vi "cameraTempControllerFrontEnd.vi"(8 "error in (no error)":errorcluster, 11 "CameraTempController":refnum<class "CameraTempController.lvclass">) -> (0 "error out":errorcluster, 3 "CameraTempController out":refnum<class "CameraTempController.lvclass">)   [LabVIEW 2009, in "Hardware.lvlib" / "Channels.lvlib" / "CameraTempController.lvclass"]
uses:
  CameraTempController.lvclass
panel:
  in  "tempControllerBackEndEvents":T1
  in  "tempControllerFrontEndEvents":T2
  out "Ready":bool
  out "Thermometer":dbl(slide)=25.0 scale=-80.0..25.0
  in  "Stop Cooling and Switch off":bool
  out "Status":string
  out "Temperature":dbl
  in  "setPoint":dbl=25.0
  # "On startup, set the desired Camera temperature set point. The Camera will then cool down to that temperature. Once reached the status field will indicate \"TEMP_STABLIZED\".\n\nAt any time you may change the setPoint to any temperature within the range of the Camera. The Camera will then warm up or cool down to that new setPoint, again indicating \"TEMP_STABLIZED\" once reached.\n\nTo Turn off the Camera temperature controller click the \"Stop\" button. This will set the temperature to 10 degrees and warm up the Camera to that temperature. At which point the temperature control program will exit.\n\nNEVER CLICK THE LABVIEW RED BUTTON TO TERMINATE THIS PROGRAM!!!!! This may cause damage to the camera! NEVER CLICK THE WINDOW CLOSE BUTTON too! This app closes itself automatically."
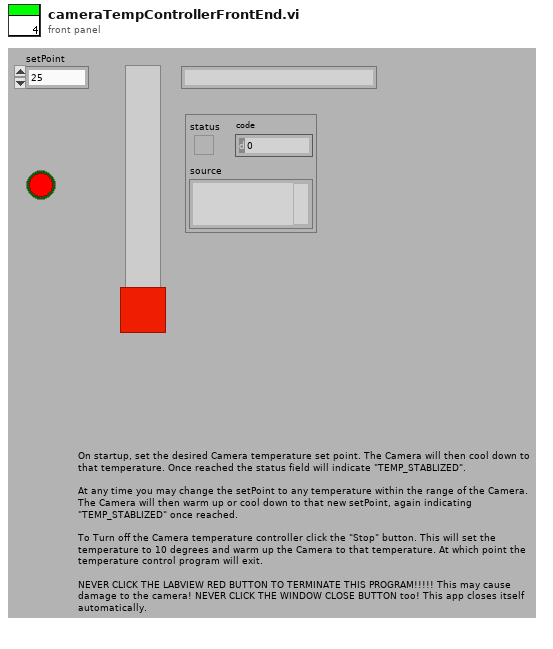
[diagram p1: front panel]
types:
  T1 = cluster{"closeEvent":refnum<user-event>, "temperatureUpdateEvent":refnum<user-event>, "displayErrorEvent":refnum<user-event>, "setPointUpdateEvent":refnum<user-event>}
  T2 = cluster{"newSetPointEvent":refnum<user-event>, "stopCoolingEvent":refnum<user-event>}
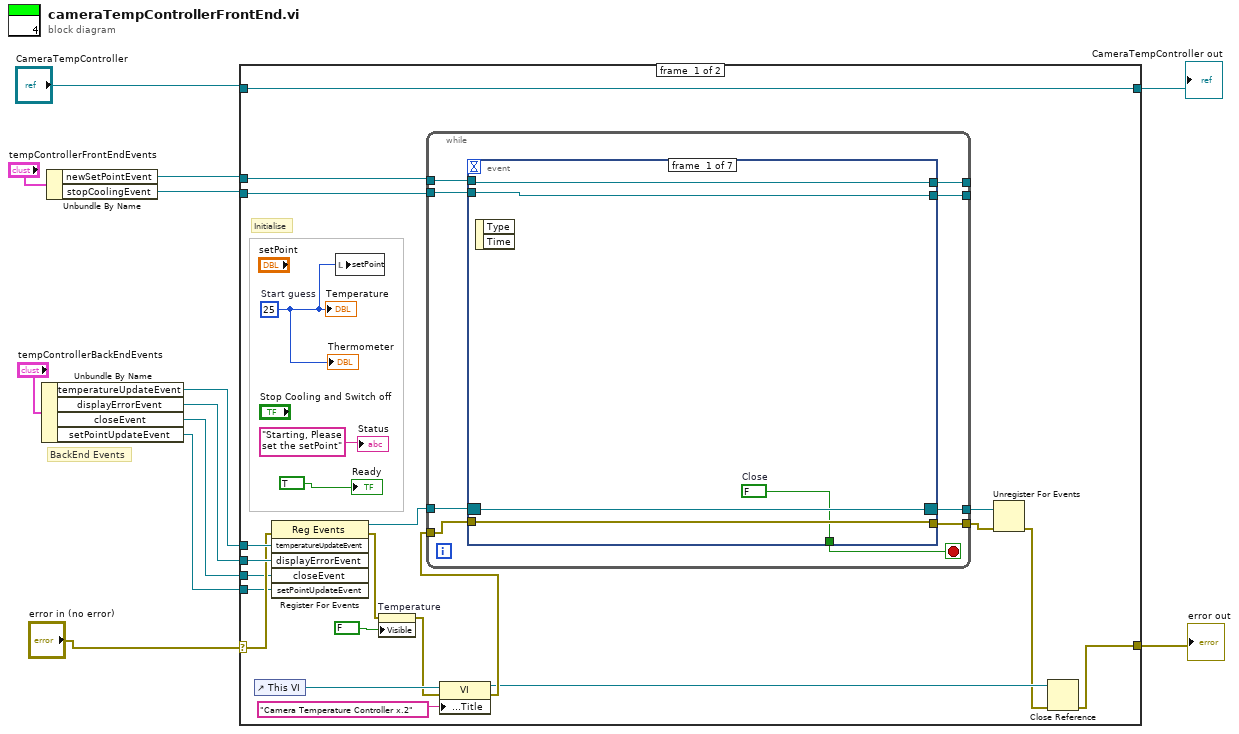
[diagram p0: block diagram]
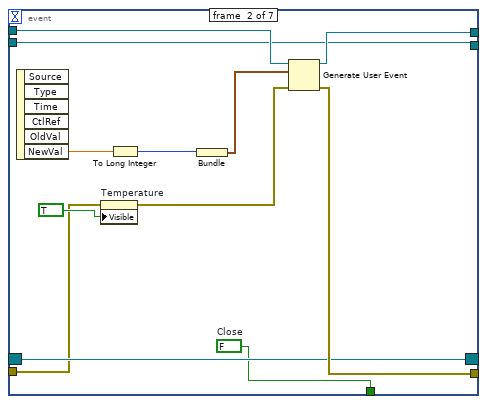
[diagram p2: hidden frame]
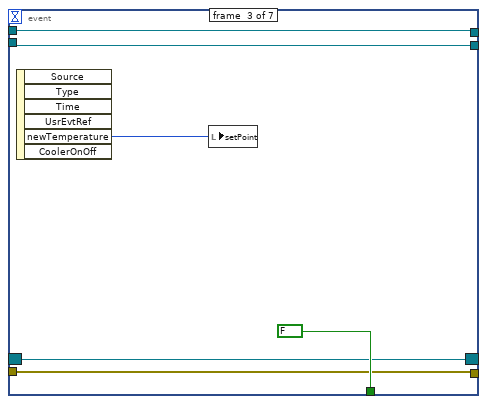
[diagram p3: hidden frame]
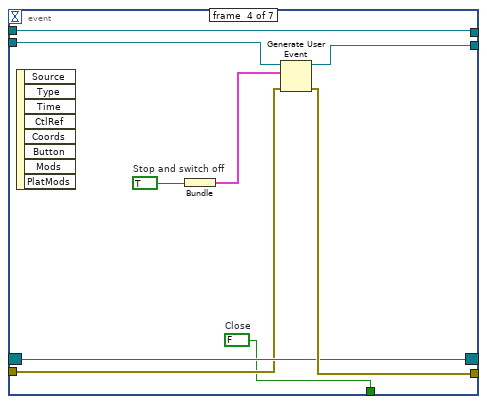
[diagram p4: hidden frame]
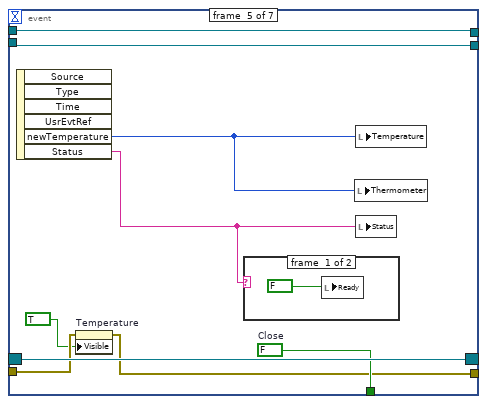
[diagram p5: hidden frame]
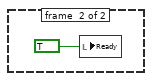
[diagram p6: hidden frame]
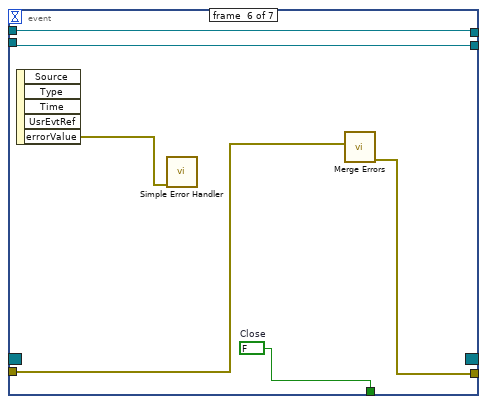
[diagram p7: hidden frame]
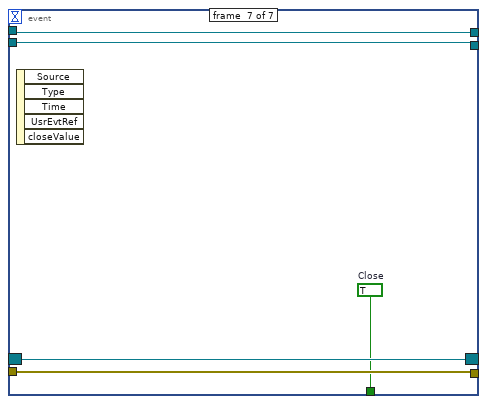
[diagram p8: hidden frame]
diagram:
  # "BackEnd Events"
  n1 = Unbundle By Name("tempControllerBackEndEvents") -> ("temperatureUpdateEvent"=w4:refnum<user-event>, "displayErrorEvent"=w3:refnum<user-event>, "closeEvent"=w2:refnum<user-event>, "setPointUpdateEvent"=w1:refnum<user-event>)
  n2 = Unbundle By Name("tempControllerFrontEndEvents") -> ("newSetPointEvent"=w7:refnum<user-event>, "stopCoolingEvent"=w6:refnum<user-event>)
  n3 = case shown="No Error" "error in (no error)" {
    selector: "error in (no error)" -> [w31 w100]
    tunnel: [w13 w100] -> w11
    tunnel: [w35 w99] -> w9
    tunnel: "CameraTempController" -> [w35 w99]
    tunnel: w6 -> [w29 _]
    tunnel: w4 -> [w33 _]
    tunnel: w3 -> [w32 _]
    tunnel: w2 -> [w28 _]
    tunnel: w1 -> [w26 _]
    tunnel: w7 -> [w23 _]
    frame #0 {
      w21 = 25  # Start guess
      # "Initialise"
      n4 = control-ref of="This VI"() -> (w19:refnum<vi>)
      n5 = register-events(error in=w31, w33, w32, w28, w26) -> (reference out=w30:refnum<event-registration>, error out=w25:errorcluster)  [unwired: 1 in]
      n6 = local write "setPoint"(w21) -> ()
      n7 = property on="Temperature" class="DigNum (strict)"(error in=w25, "Visible"=FALSE) -> (error out=w18:errorcluster)  [unwired: 1 in, 1 out]
      n8 = property class="VI"(reference=w19, error in=w18, "Front Panel.Title"="Camera Temperature Controller x.2") -> (reference out=w15:refnum<vi>, error out=w17:errorcluster)
      n9 = while {
        tunnel: [w44] -> w34
        tunnel: w30 -> [w43]
        tunnel: w23 -> [w42]
        tunnel: w29 -> [w41]
        tunnel: w17 -> [w40]
        tunnel: [w39] -> _
        tunnel: [w38] -> w22
        tunnel: [w37] -> _
        stop <- w36 stop-if-true
        n10 = event shown="[1] \"setPoint\": Value Change" {
          selector: w43 -> [w49 w58 w64 w73 w82 _ w97]
          dyn-events: [w49 w58 w64 w73 w82 _ w97] -> w44
          timeout: _ -> [_ _ _ _ _ _ _]
          tunnel: w42 -> [w47 w55 w63 w70 w84 w92 w95]
          tunnel: w41 -> [w46 w54 w62 w76 w83 w90 w96]
          tunnel: w40 -> [w48 w51 w65 w72 w80 w88 w98]
          tunnel: [w47 w60 w63 w70 w84 w92 w95] -> w39
          tunnel: [w48 w59 w65 w74 w79 w93 w98] -> w38
          tunnel: [w46 w54 w62 w75 w83 w90 w96] -> w37
          tunnel: [w45 w57 FALSE w68 w81 w91 w94] -> w36
          event #0 {
            w45 = FALSE  # Close
            n11 = event-data() -> ()  [unwired: 1 in, 2 out]
          }
          event #1 {
            w57 = FALSE  # Close
            n12 = event-data() -> ("NewVal"=w61:dbl)  [unwired: 1 in, 5 out]
            n13 = property on="Temperature" class="DigNum (strict)"(error in=w51, "Visible"=TRUE) -> (error out=w50:errorcluster)  [unwired: 1 in, 1 out]
            n14 = To Long Integer(number=w61) -> (32bit integer=w56:i32)
            n15 = Bundle(w56) -> (w53:cluster{i32})  [unwired: 1 in]
            n16 = Generate User Event(user event=w55, event data cluster=w53, error in=w50) -> (user event out=w60:refnum<user-event>, error out=w59:errorcluster)
          }
          event #2 {
            n17 = event-data() -> ("newTemperature"=w67:i32)  [unwired: 1 in, 5 out]
            n18 = local write "setPoint"(w67) -> ()
          }
          event #3 {
            w68 = FALSE  # Close
            w69 = TRUE  # Stop and switch off
            n19 = event-data() -> ()  [unwired: 1 in, 8 out]
            n20 = Bundle("Stop and switch off"=w69) -> (w71:cluster{"Stop and switch off":bool})  [unwired: 1 in]
            n21 = Generate User Event(user event=w76, event data cluster=w71, error in=w72) -> (user event out=w75:refnum<user-event>, error out=w74:errorcluster)
          }
          event #4 {
            w81 = FALSE  # Close
            n22 = event-data() -> ("newTemperature"=w85:i32, "Status"=w77:string)  [unwired: 1 in, 4 out]
            n23 = property on="Temperature" class="DigNum (strict)"(error in=w80, "Visible"=TRUE) -> (error out=w79:errorcluster)  [unwired: 1 in, 1 out]
            n24 = case shown="\"TEMP_STABILIZED\"" w77 {
              frame #0 {
                n25 = local write "Ready"(FALSE) -> ()
              }
              frame #1 {
                n26 = local write "Ready"(TRUE) -> ()
              }
            }
            n27 = local write "Thermometer"(w85) -> ()
            n28 = local write "Temperature"(w85) -> ()
            n29 = local write "Status"(w77) -> ()
          }
          event #5 {
            w91 = FALSE  # Close
            n30 = event-data() -> ("errorValue"=w89:errorcluster)  [unwired: 1 in, 4 out]
            n31 = call <vilib>:"Simple Error Handler.vi"("error in (no error)"=w89) -> ()  [unwired: 4 in, 5 out]
            n32 = call <vilib>:"Merge Errors.vi"("error in 2 (no error)"=w88) -> ("error out"=w93:errorcluster)  [unwired: 6 in]
          }
          event #6 {
            w94 = TRUE  # Close
            n33 = event-data() -> ()  [unwired: 1 in, 5 out]
          }
        }
      }
      n34 = Unregister For Events(event registration refnum=w34, error in=w22) -> (error out=w14:errorcluster)
      n35 = Close Reference(reference=w15, error in (no error)=w14) -> (error out=w13:errorcluster)
      "Status" <- "Starting, Please set the setPoint"
      "Ready" <- TRUE
      "Temperature" <- w21
      "Thermometer" <- w21
    }
    frame #1 {
    }
  }
  "error out" <- w11
  "CameraTempController out" <- w9
